vi "Dresden R2R Sputter 03.02.2018 IY24.vi"() -> ()   [LabVIEW 2009] (continued)
                                }
                                frame #1 {
                                }
                                }
                                }
                                frame #1 {
                                n25584 = local read "Semi"() -> (w30862:bool)
                                n25585 = case shown="False" w30862 {
                                frame #0 {
                                n25586 = while {
                                i -> [w30872]
                                stop <- w30863 stop-if-true
                                n25587 = Greater Or Equal?(x=w30872, y=240) -> (x >= y?=w30871:bool)
                                n25588 = case shown="True" w30871 {
                                frame #0 {
                                }
                                frame #1 {
                                n25589 = local write "Semi"(TRUE ("Semi")) -> ()
                                }
                                }
                                n25590 = local read "Set DC Power       :"() -> (w30868:dbl)
                                n25591 = local read "Actual DC Power"() -> (w30867:dbl)
                                n25592 = Subtract(x=w30868, y=w30867) -> (x-y=w30870:dbl)
                                n25593 = Less?(x=w30870, y=10.0) -> (x < y?=w30865:bool)
                                n25594 = local read "Semi"() -> (w30864:bool)
                                n25595 = Or(x=w30865, y=w30864) -> (x .or. y?=w30863:bool)
                                n25596 = Wait Until Next ms Multiple(millisecond multiple=u32 500) -> ()  [unwired: 1 out]
                                }
                                }
                                frame #1 {
                                }
                                }
                                }
                                }
                                }
                                frame #3 {
                                # "Set Pressure for coating"
                                n25597 = stacked-sequence {
                                frame #0 {
                                n25598 = local read "Semi"() -> (w30875:bool)
                                n25599 = case shown="False" w30875 {
                                frame #0 {
                                n25600 = stacked-sequence {
                                frame #0 {
                                n25601 = local read "Semi"() -> (w30876:bool)
                                n25602 = case shown="False" w30876 {
                                frame #0 {
                                n25603 = local read "R Set Pressure mtorr"() -> (w30877:dbl)
                                n25604 = local write "Set_pressure_value 2"(w30877) -> ()
                                }
                                frame #1 {
                                }
                                }
                                }
                                frame #1 {
                                n25605 = local read "Semi"() -> (w30878:bool)
                                n25606 = case shown="False" w30878 {
                                frame #0 {
                                n25607 = Wait (ms)(milliseconds to wait=u32 200) -> ()  [unwired: 1 out]
                                }
                                frame #1 {
                                }
                                }
                                }
                                frame #2 {
                                n25608 = local read "Semi"() -> (w30880:bool)
                                n25609 = case shown="False" w30880 {
                                frame #0 {
                                n25610 = local write "Pc_bv2_auto_set_pressure"(TRUE ("Pc_bv1_auto_set_pressure")) -> ()
                                }
                                frame #1 {
                                }
                                }
                                }
                                frame #3 {
                                n25611 = local read "Semi"() -> (w30882:bool)
                                n25612 = case shown="False" w30882 {
                                frame #0 {
                                n25613 = while {
                                i -> [w30893]
                                stop <- w30885 stop-if-true
                                n25614 = local read "Set_pressure_value 2"() -> (w30883:dbl)
                                n25615 = Greater?(x=w30893, y=300) -> (0:w30887:bool)
                                n25616 = Add(x=1.0, y=w30883) -> (x+y=w30889:dbl)
                                n25617 = Subtract(x=w30883, y=1.0) -> (x-y=w30890:dbl)
                                n25618 = local read "Pressure 2"() -> (w30884:i32)
                                n25619 = In Range and Coerce(upper limit=w30889, x=w30884, lower limit=w30890) -> (In Range?=w30888:bool)  [unwired: 1 out]
                                n25620 = case shown="False" w30888 {
                                tunnel: [FALSE TRUE] -> w30886
                                frame #0 {
                                n25621 = Wait Until Next ms Multiple(millisecond multiple=u32 200) -> ()  [unwired: 1 out]
                                }
                                frame #1 {
                                }
                                }
                                n25622 = Or(x=w30886, y=w30887) -> (x .or. y?=w30885:bool)
                                }
                                }
                                frame #1 {
                                }
                                }
                                }
                                frame #4 {
                                n25623 = local read "Semi"() -> (w30898:bool)
                                n25624 = case shown="False" w30898 {
                                frame #0 {
                                n25625 = local read "Set_pressure_value 2"() -> (w30899:dbl)
                                n25626 = Add(x=1.0, y=w30899) -> (x+y=w30902:dbl)
                                n25627 = Subtract(x=w30899, y=1.0) -> (x-y=w30903:dbl)
                                n25628 = local read "Pressure 2"() -> (w30900:i32)
                                n25629 = In Range and Coerce(upper limit=w30902, x=w30900, lower limit=w30903) -> (In Range?=w30901:bool)  [unwired: 1 out]
                                n25630 = case shown="False" w30901 {
                                frame #0 {
                                n25631 = local read "R Set Pressure mtorr"() -> (w30906:dbl)
                                n25632 = local write "Set_pressure_value 2"(w30906) -> ()
                                }
                                frame #1 {
                                }
                                }
                                }
                                frame #1 {
                                }
                                }
                                }
                                frame #5 {
                                n25633 = local read "Semi"() -> (w30907:bool)
                                n25634 = case shown="False" w30907 {
                                frame #0 {
                                n25635 = local read "Set_pressure_value 2"() -> (w30908:dbl)
                                n25636 = Add(x=1.0, y=w30908) -> (x+y=w30911:dbl)
                                n25637 = Subtract(x=w30908, y=1.0) -> (x-y=w30912:dbl)
                                n25638 = local read "Pressure 2"() -> (w30909:i32)
                                n25639 = In Range and Coerce(upper limit=w30911, x=w30909, lower limit=w30912) -> (In Range?=w30910:bool)  [unwired: 1 out]
                                n25640 = case shown="False" w30910 {
                                frame #0 {
                                n25641 = local write "Pc_bv2_auto_set_pressure"(TRUE ("Pc_bv1_auto_set_pressure")) -> ()
                                }
                                frame #1 {
                                }
                                }
                                }
                                frame #1 {
                                }
                                }
                                }
                                frame #6 {
                                n25642 = local read "Semi"() -> (w30916:bool)
                                n25643 = case shown="False" w30916 {
                                frame #0 {
                                n25644 = while {
                                i -> [w30927]
                                stop <- w30918 stop-if-true
                                n25645 = local read "Set_pressure_value 2"() -> (w30922:dbl)
                                n25646 = Greater?(x=w30927, y=300) -> (0:w30920:bool)
                                n25647 = Add(x=1.0, y=w30922) -> (x+y=w30923:dbl)
                                n25648 = Subtract(x=w30922, y=1.0) -> (x-y=w30924:dbl)
                                n25649 = local read "Pressure 2"() -> (w30917:i32)
                                n25650 = In Range and Coerce(upper limit=w30923, x=w30917, lower limit=w30924) -> (In Range?=w30921:bool)  [unwired: 1 out]
                                n25651 = case shown="False" w30921 {
                                tunnel: [FALSE TRUE] -> w30919
                                frame #0 {
                                n25652 = Wait Until Next ms Multiple(millisecond multiple=u32 200) -> ()  [unwired: 1 out]
                                }
                                frame #1 {
                                }
                                }
                                n25653 = Or(x=w30919, y=w30920) -> (x .or. y?=w30918:bool)
                                }
                                }
                                frame #1 {
                                }
                                }
                                }
                                frame #7 {
                                n25654 = local read "Semi"() -> (w30932:bool)
                                n25655 = case shown="False" w30932 {
                                frame #0 {
                                n25656 = local read "Set_pressure_value 2"() -> (w30935:dbl)
                                n25657 = Add(x=1.0, y=w30935) -> (x+y=w30936:dbl)
                                n25658 = Subtract(x=w30935, y=1.0) -> (x-y=w30937:dbl)
                                n25659 = local read "Pressure 2"() -> (w30933:i32)
                                n25660 = In Range and Coerce(upper limit=w30936, x=w30933, lower limit=w30937) -> (In Range?=w30934:bool)  [unwired: 1 out]
                                n25661 = case shown="False" w30934 {
                                frame #0 {
                                n25662 = local write "Semi"(TRUE ("Semi")) -> ()
                                n25663 = local write "Error Message"("Coating Pressure could not be adjusted !" ("Error Message")) -> ()
                                }
                                frame #1 {
                                }
                                }
                                }
                                frame #1 {
                                }
                                }
                                }
                                }
                                }
                                frame #1 {
                                }
                                }
                                }
                                frame #1 {
                                n25664 = local read "Semi"() -> (w30942:bool)
                                n25665 = case shown="False" w30942 {
                                frame #0 {
                                n25666 = local write "SDC1 9"(TRUE ("SDC1 9")) -> ()
                                n25667 = Wait (ms)(milliseconds to wait=u32 1000) -> ()  [unwired: 1 out]
                                }
                                frame #1 {
                                }
                                }
                                }
                                }
                                }
                                }
                                }
                                frame #1 {
                                }
                                }
                                }
                                frame #11 {
                                n25668 = local read "Semi"() -> (w30945:bool)
                                n25669 = case shown="False" w30945 {
                                frame #0 {
                                n25670 = local write "Start_roll"(TRUE ("Start_roll")) -> ()
                                n25671 = Wait (ms)(milliseconds to wait=u32 300) -> ()  [unwired: 1 out]
                                }
                                frame #1 {
                                }
                                }
                                }
                                frame #12 {
                                n25672 = local read "Semi"() -> (w30948:bool)
                                n25673 = case shown="False" w30948 {
                                frame #0 {
                                n25674 = stacked-sequence {
                                frame #0 {
                                n25675 = local read "R Single DC Step1 Coating Power Active"() -> (w30949:bool)
                                n25676 = case shown="True" w30949 {
                                frame #0 {
                                }
                                frame #1 {
                                n25677 = while {
                                stop <- w30951 stop-if-true
                                n25678 = local read "R Single DC Interval length"() -> (w30955:dbl)
                                n25679 = local read "Actual Length"() -> (w30954:dbl)
                                n25680 = Greater Or Equal?(x=w30954, y=w30955) -> (x >= y?=w30953:bool)
                                n25681 = local read "Semi"() -> (w30952:bool)
                                n25682 = Or(x=w30953, y=w30952) -> (x .or. y?=w30951:bool)
                                n25683 = Wait Until Next ms Multiple(millisecond multiple=u32 300) -> ()  [unwired: 1 out]
                                }
                                }
                                }
                                }
                                frame #1 {
                                n25684 = local read "R Single DC Step2 Coating Power Active"() -> (w30956:bool)
                                n25685 = case shown="True" w30956 {
                                frame #0 {
                                }
                                frame #1 {
                                n25686 = stacked-sequence {
                                frame #0 {
                                n25687 = local read "Semi"() -> (w30957:bool)
                                n25688 = case shown="False" w30957 {
                                frame #0 {
                                n25689 = local read "R Single DC Step2 Coating Power"() -> (w30959:dbl)
                                n25690 = Wait (ms)(milliseconds to wait=u32 200) -> ()  [unwired: 1 out]
                                n25691 = local write "Set DC Power       :"(w30959) -> ()
                                }
                                frame #1 {
                                }
                                }
                                }
                                frame #1 {
                                n25692 = local read "Semi"() -> (w30960:bool)
                                n25693 = case shown="False" w30960 {
                                frame #0 {
                                n25694 = local write "Dc_auto_set"(TRUE ("Dc_auto_set")) -> ()
                                }
                                frame #1 {
                                }
                                }
                                }
                                frame #2 {
                                n25695 = while {
                                stop <- w30966 stop-if-true
                                n25696 = local read "R Single DC Interval length"() -> (w30965:dbl)
                                n25697 = local read "Actual Length"() -> (w30969:dbl)
                                n25698 = Multiply(x=w30965, y=2.0) -> (x*y=w30963:dbl)
                                n25699 = Greater Or Equal?(x=w30969, y=w30963) -> (x >= y?=w30968:bool)
                                n25700 = local read "Semi"() -> (w30967:bool)
                                n25701 = Or(x=w30968, y=w30967) -> (x .or. y?=w30966:bool)
                                n25702 = Wait Until Next ms Multiple(millisecond multiple=u32 300) -> ()  [unwired: 1 out]
                                }
                                }
                                }
                                }
                                }
                                }
                                frame #2 {
                                n25703 = local read "R Single DC Step3 Coating Power Active"() -> (w30970:bool)
                                n25704 = case shown="True" w30970 {
                                frame #0 {
                                }
                                frame #1 {
                                n25705 = stacked-sequence {
                                frame #0 {
                                n25706 = local read "Semi"() -> (w30971:bool)
                                n25707 = case shown="False" w30971 {
                                frame #0 {
                                n25708 = local read "R Single DC Step3 Coating Power"() -> (w30973:dbl)
                                n25709 = Wait (ms)(milliseconds to wait=u32 200) -> ()  [unwired: 1 out]
                                n25710 = local write "Set DC Power       :"(w30973) -> ()
                                }
                                frame #1 {
                                }
                                }
                                }
                                frame #1 {
                                n25711 = local read "Semi"() -> (w30974:bool)
                                n25712 = case shown="False" w30974 {
                                frame #0 {
                                n25713 = local write "Dc_auto_set"(TRUE ("Dc_auto_set")) -> ()
                                }
                                frame #1 {
                                }
                                }
                                }
                                frame #2 {
                                n25714 = while {
                                stop <- w30980 stop-if-true
                                n25715 = local read "R Single DC Interval length"() -> (w30979:dbl)
                                n25716 = local read "Actual Length"() -> (w30983:dbl)
                                n25717 = Multiply(x=w30979, y=3.0) -> (x*y=w30977:dbl)
                                n25718 = Greater Or Equal?(x=w30983, y=w30977) -> (x >= y?=w30982:bool)
                                n25719 = local read "Semi"() -> (w30981:bool)
                                n25720 = Or(x=w30982, y=w30981) -> (x .or. y?=w30980:bool)
                                n25721 = Wait Until Next ms Multiple(millisecond multiple=u32 300) -> ()  [unwired: 1 out]
                                }
                                }
                                }
                                }
                                }
                                }
                                frame #3 {
                                n25722 = local read "R Single DC Step4 Coating Power Active"() -> (w30984:bool)
                                n25723 = case shown="True" w30984 {
                                frame #0 {
                                }
                                frame #1 {
                                n25724 = stacked-sequence {
                                frame #0 {
                                n25725 = local read "Semi"() -> (w30985:bool)
                                n25726 = case shown="False" w30985 {
                                frame #0 {
                                n25727 = local read "R Single DC Step4 Coating Power"() -> (w30987:dbl)
                                n25728 = Wait (ms)(milliseconds to wait=u32 200) -> ()  [unwired: 1 out]
                                n25729 = local write "Set DC Power       :"(w30987) -> ()
                                }
                                frame #1 {
                                }
                                }
                                }
                                frame #1 {
                                n25730 = local read "Semi"() -> (w30988:bool)
                                n25731 = case shown="False" w30988 {
                                frame #0 {
                                n25732 = local write "Dc_auto_set"(TRUE ("Dc_auto_set")) -> ()
                                }
                                frame #1 {
                                }
                                }
                                }
                                frame #2 {
                                n25733 = while {
                                stop <- w30994 stop-if-true
                                n25734 = local read "R Single DC Interval length"() -> (w30993:dbl)
                                n25735 = local read "Actual Length"() -> (w30997:dbl)
                                n25736 = Multiply(x=w30993, y=4.0) -> (x*y=w30991:dbl)
                                n25737 = Greater Or Equal?(x=w30997, y=w30991) -> (x >= y?=w30996:bool)
                                n25738 = local read "Semi"() -> (w30995:bool)
                                n25739 = Or(x=w30996, y=w30995) -> (x .or. y?=w30994:bool)
                                n25740 = Wait Until Next ms Multiple(millisecond multiple=u32 300) -> ()  [unwired: 1 out]
                                }
                                }
                                }
                                }
                                }
                                }
                                frame #4 {
                                n25741 = local read "R Single DC Step5 Coating Power Active"() -> (w30998:bool)
                                n25742 = case shown="True" w30998 {
                                frame #0 {
                                }
                                frame #1 {
                                n25743 = stacked-sequence {
                                frame #0 {
                                n25744 = local read "Semi"() -> (w30999:bool)
                                n25745 = case shown="False" w30999 {
                                frame #0 {
                                n25746 = local read "R Single DC Step5 Coating Power"() -> (w31001:dbl)
                                n25747 = Wait (ms)(milliseconds to wait=u32 200) -> ()  [unwired: 1 out]
                                n25748 = local write "Set DC Power       :"(w31001) -> ()
                                }
                                frame #1 {
                                }
                                }
                                }
                                frame #1 {
                                n25749 = local read "Semi"() -> (w31002:bool)
                                n25750 = case shown="False" w31002 {
                                frame #0 {
                                n25751 = local write "Dc_auto_set"(TRUE ("Dc_auto_set")) -> ()
                                }
                                frame #1 {
                                }
                                }
                                }
                                frame #2 {
                                n25752 = while {
                                stop <- w31008 stop-if-true
                                n25753 = local read "R Single DC Interval length"() -> (w31007:dbl)
                                n25754 = local read "Actual Length"() -> (w31011:dbl)
                                n25755 = Multiply(x=w31007, y=5.0) -> (x*y=w31005:dbl)
                                n25756 = Greater Or Equal?(x=w31011, y=w31005) -> (x >= y?=w31010:bool)
                                n25757 = local read "Semi"() -> (w31009:bool)
                                n25758 = Or(x=w31010, y=w31009) -> (x .or. y?=w31008:bool)
                                n25759 = Wait Until Next ms Multiple(millisecond multiple=u32 300) -> ()  [unwired: 1 out]
                                }
                                }
                                }
                                }
                                }
                                }
                                }
                                }
                                frame #1 {
                                }
                                }
                                }
                                frame #13 {
                                n25760 = local read "Semi"() -> (w31012:bool)
                                n25761 = case shown="False" w31012 {
                                frame #0 {
                                n25762 = local write "SDC1 13b"(TRUE ("SDC1 13b")) -> ()
                                n25763 = Wait (ms)(milliseconds to wait=u32 1000) -> ()  [unwired: 1 out]
                                }
                                frame #1 {
                                }
                                }
                                }
                                }
                                }
                                frame #1 {
                                }
                                }
                                }
                                frame #17 {
                                # "encoder info  add to other web selection"
                                n25764 = stacked-sequence {
                                frame #0 {
                                n25765 = local read "Semi"() -> (w31015:bool)
                                n25766 = case shown="False" w31015 {
                                frame #0 {
                                # "salinim hareketi"
                                n25767 = local read "R_Web_selection"() -> (w31016:enum32{"Web", "Other"})
                                n25768 = case shown="\"Other\"" w31016 {
                                frame #0 {
                                # "TC -ROLL"
                                }
                                frame #1 {
                                n25769 = disable-structure shown="Disabled" {
                                frame #0 {
                                # "OTHER"
                                n25770 = local read "Semi"() -> (w31017:bool)
                                n25771 = case shown="False" w31017 {
                                frame #0 {
                                n25772 = stacked-sequence {
                                frame #0 {
                                n25773 = local read "Semi"() -> (w31018:bool)
                                n25774 = case shown="False" w31018 {
                                frame #0 {
                                n25775 = stacked-sequence {
                                frame #0 {
                                n25776 = local read "Semi"() -> (w31019:bool)
                                n25777 = case shown="False" w31019 {
                                frame #0 {
                                n25778 = while {
                                i -> [w31022]
                                stop <- w31023 stop-if-true
                                n25779 = Greater?(x=w31022, y=300) -> (0:w31020:bool)
                                n25780 = case shown="True" w31020 {
                                frame #0 {
                                }
                                frame #1 {
                                n25781 = local write "Semi"(TRUE ("Semi")) -> ()
                                }
                                }
                                n25782 = local read "RC_13"() -> (w31026:bool)
                                n25783 = case shown="False" w31026 {
                                tunnel: [FALSE ("ch2_1") TRUE ("ch2_1")] -> w31025
                                frame #0 {
                                n25784 = local write "Routine_check_transfer"(TRUE ("ch2_1")) -> ()
                                n25785 = Wait Until Next ms Multiple(millisecond multiple=u32 1000) -> ()  [unwired: 1 out]
                                }
                                frame #1 {
                                }
                                }
                                n25786 = local read "Semi"() -> (w31024:bool)
                                n25787 = Or(x=w31025, y=w31024) -> (x .or. y?=w31023:bool)
                                }
                                }
                                frame #1 {
                                }
                                }
                                }
                                frame #1 {
                                n25788 = local read "Semi"() -> (w31032:bool)
                                n25789 = case shown="False" w31032 {
                                frame #0 {
                                n25790 = while {
                                i -> [w31039]
                                stop <- w31034 stop-if-true
                                n25791 = Greater?(x=w31039, y=100) -> (0:w31037:bool)
                                n25792 = case shown="True" w31037 {
                                frame #0 {
                                }
                                frame #1 {
                                n25793 = local write "Error Message"("Transfer process was cancelled.\nPlease check GV connections." ("Error Message")) -> ()
                                n25794 = local write "Semi"(TRUE ("Semi")) -> ()
                                }
                                }
                                n25795 = local read "Ch1_Trns_interlock_di"() -> (w31033:bool)
                                n25796 = case shown="False" w31033 {
                                tunnel: [w31041 TRUE] -> w31036
                                frame #0 {
                                n25797 = local read "Ch1_TGV_control_di"() -> (w31040:bool)
                                n25798 = case shown="False" w31040 {
                                tunnel: [FALSE TRUE] -> w31041
                                frame #0 {
                                n25799 = Wait Until Next ms Multiple(millisecond multiple=u32 50) -> ()  [unwired: 1 out]
                                n25800 = local write "Ch1_TGV_control_do"(TRUE ("Ch1_pet_cool_up_do")) -> ()
                                }
                                frame #1 {
                                }
                                }
                                }
                                frame #1 {
                                }
                                }
                                n25801 = local read "Semi"() -> (w31035:bool)
                                n25802 = Or(x=w31036, y=w31035) -> (x .or. y?=w31034:bool)
                                }
                                }
                                frame #1 {
                                }
                                }
                                }
                                frame #2 {
                                n25803 = local read "Semi"() -> (w31049:bool)
                                n25804 = case shown="False" w31049 {
                                frame #0 {
                                n25805 = while {
                                i -> [w31056]
                                stop <- w31051 stop-if-true
                                n25806 = Greater?(x=w31056, y=100) -> (0:w31054:bool)
                                n25807 = case shown="True" w31054 {
                                frame #0 {
                                }
                                frame #1 {
                                n25808 = local write "Error Message"("Transfer process was cancelled.\nPlease check GV connections." ("Error Message")) -> ()
                                n25809 = local write "Semi"(TRUE ("Semi")) -> ()
                                }
                                }
                                n25810 = local read "Ch2_Trns_interlock_di"() -> (w31050:bool)
                                n25811 = case shown="False" w31050 {
                                tunnel: [w31058 TRUE] -> w31053
                                frame #0 {
                                n25812 = local read "Ch2_TGV_control_di"() -> (w31057:bool)
                                n25813 = case shown="False" w31057 {
                                tunnel: [FALSE TRUE] -> w31058
                                frame #0 {
                                n25814 = Wait Until Next ms Multiple(millisecond multiple=u32 50) -> ()  [unwired: 1 out]
                                n25815 = local write "Ch2_TGV_control_do"(TRUE ("Ch1_pet_cool_up_do")) -> ()
                                }
                                frame #1 {
                                }
                                }
                                }
                                frame #1 {
                                }
                                }
                                n25816 = local read "Semi"() -> (w31052:bool)
                                n25817 = Or(x=w31053, y=w31052) -> (x .or. y?=w31051:bool)
                                }
                                }
                                frame #1 {
                                }
                                }
                                }
                                frame #3 {
                                n25818 = local read "Semi"() -> (w31066:bool)
                                n25819 = case shown="False" w31066 {
                                frame #0 {
                                n25820 = while {
                                i -> [w31073]
                                stop <- w31068 stop-if-true
                                n25821 = Greater?(x=w31073, y=100) -> (0:w31071:bool)
                                n25822 = case shown="True" w31071 {
                                frame #0 {
                                }
                                frame #1 {
                                n25823 = local write "Error Message"("Transfer process was cancelled.\nPlease check GV connections." ("Error Message")) -> ()
                                n25824 = local write "Semi"(TRUE ("Semi")) -> ()
                                }
                                }
                                n25825 = local read "Ch3_Trns_interlock_di"() -> (w31067:bool)
                                n25826 = case shown="False" w31067 {
                                tunnel: [w31075 TRUE] -> w31070
                                frame #0 {
                                n25827 = local read "Ch3_TGV_control_di"() -> (w31074:bool)
                                n25828 = case shown="False" w31074 {
                                tunnel: [FALSE TRUE] -> w31075
                                frame #0 {
                                n25829 = Wait Until Next ms Multiple(millisecond multiple=u32 50) -> ()  [unwired: 1 out]
                                n25830 = local write "Ch3_TGV_control_do"(TRUE ("Ch1_pet_cool_up_do")) -> ()
                                }
                                frame #1 {
                                }
                                }
                                }
                                frame #1 {
                                }
                                }
                                n25831 = local read "Semi"() -> (w31069:bool)
                                n25832 = Or(x=w31070, y=w31069) -> (x .or. y?=w31068:bool)
                                }
                                }
                                frame #1 {
                                }
                                }
                                }
                                frame #4 {
                                n25833 = local read "Semi"() -> (w31083:bool)
                                n25834 = case shown="False" w31083 {
                                frame #0 {
                                n25835 = while {
                                i -> [w31090]
                                stop <- w31085 stop-if-true
                                n25836 = Greater?(x=w31090, y=100) -> (0:w31088:bool)
                                n25837 = case shown="True" w31088 {
                                frame #0 {
                                }
                                frame #1 {
                                n25838 = local write "Error Message"("Transfer process was cancelled.\nPlease check GV connections." ("Error Message")) -> ()
                                n25839 = local write "Semi"(TRUE ("Semi")) -> ()
                                }
                                }
                                n25840 = local read "Ch3_Trns_interlock_di"() -> (w31084:bool)
                                n25841 = case shown="False" w31084 {
                                tunnel: [w31092 TRUE] -> w31087
                                frame #0 {
                                n25842 = local read "Ch3_TGV_control_di"() -> (w31091:bool)
                                n25843 = case shown="False" w31091 {
                                tunnel: [FALSE TRUE] -> w31092
                                frame #0 {
                                n25844 = Wait Until Next ms Multiple(millisecond multiple=u32 50) -> ()  [unwired: 1 out]
                                n25845 = local write "Ch3_TGV_control_do"(TRUE ("Ch1_pet_cool_up_do")) -> ()
                                }
                                frame #1 {
                                }
                                }
                                }
                                frame #1 {
                                }
                                }
                                n25846 = local read "Semi"() -> (w31086:bool)
                                n25847 = Or(x=w31087, y=w31086) -> (x .or. y?=w31085:bool)
                                }
                                }
                                frame #1 {
                                }
                                }
                                }
                                frame #5 {
                                n25848 = local read "Semi"() -> (w31100:bool)
                                n25849 = case shown="False" w31100 {
                                frame #0 {
                                n25850 = while {
                                i -> [w31103]
                                stop <- w31104 stop-if-true
                                n25851 = Greater?(x=w31103, y=50) -> (0:w31101:bool)
                                n25852 = case shown="True" w31101 {
                                frame #0 {
                                }
                                frame #1 {
                                n25853 = local write "Error Message"("Transfer process was\ncancelled.Please check right slow sensor." ("Error Message")) -> ()
                                n25854 = local write "Semi"(TRUE ("Semi")) -> ()
                                }
                                }
                                n25855 = local read "Cnt_Right_slow_di"() -> (w31107:bool)
                                n25856 = case shown="False" w31107 {
                                tunnel: [FALSE ("Ch1_pet_cool_up_do") TRUE ("Ch1_pet_cool_up_do")] -> w31106
                                frame #0 {
                                n25857 = local write "Cnt_Right_slow_do"(TRUE ("Ch1_pet_cool_up_do")) -> ()
                                n25858 = Wait Until Next ms Multiple(millisecond multiple=u32 200) -> ()  [unwired: 1 out]
                                }
                                frame #1 {
                                }
                                }
                                n25859 = local read "Semi"() -> (w31105:bool)
                                n25860 = Or(x=w31106, y=w31105) -> (x .or. y?=w31104:bool)
                                }
                                }
                                frame #1 {
                                }
                                }
                                }
                                frame #6 {
                                n25861 = local read "Semi"() -> (w31114:bool)
                                n25862 = case shown="False" w31114 {
                                frame #0 {
                                n25863 = while {
                                i -> [w31115]
                                stop <- w31119 stop-if-true
                                n25864 = Greater?(x=w31115, y=50) -> (0:w31117:bool)
                                n25865 = case shown="True" w31117 {
                                frame #0 {
                                }
                                frame #1 {
                                n25866 = local write "Error Message"("Transfer process was\ncancelled.Please check right limit sensor." ("Error Message")) -> ()
                                n25867 = local write "Semi"(TRUE ("Semi")) -> ()
                                }
                                }
                                n25868 = local read "Cnt_Right_limit_di"() -> (w31121:bool)
                                n25869 = case shown="False" w31121 {
                                tunnel: [FALSE ("Ch1_pet_cool_up_do") TRUE ("Ch1_pet_cool_up_do")] -> w31120
                                frame #0 {
                                n25870 = local write "Cnt_Right_limit_do"(TRUE ("Ch1_pet_cool_up_do")) -> ()
                                n25871 = Wait Until Next ms Multiple(millisecond multiple=u32 200) -> ()  [unwired: 1 out]
                                }
                                frame #1 {
                                }
                                }
                                n25872 = local read "Semi"() -> (w31118:bool)
                                n25873 = Or(x=w31120, y=w31118) -> (x .or. y?=w31119:bool)
                                }
                                }
                                frame #1 {
                                }
                                }
                                }
                                frame #7 {
                                n25874 = local read "Semi"() -> (w31128:bool)
                                n25875 = case shown="False" w31128 {
                                frame #0 {
                                n25876 = while {
                                i -> [w31131]
                                stop <- w31132 stop-if-true
                                n25877 = Greater?(x=w31131, y=50) -> (0:w31129:bool)
                                n25878 = case shown="True" w31129 {
                                frame #0 {
                                }
                                frame #1 {
                                n25879 = local write "Error Message"("Transfer process was\ncancelled.Please check left slow sensor." ("Error Message")) -> ()
                                n25880 = local write "Semi"(TRUE ("Semi")) -> ()
                                }
                                }
                                n25881 = local read "Cnt_Left_slow_di"() -> (w31135:bool)
                                n25882 = case shown="False" w31135 {
                                tunnel: [FALSE ("Ch1_pet_cool_up_do") TRUE ("Ch1_pet_cool_up_do")] -> w31134
                                frame #0 {
                                n25883 = local write "Cnt_Left_slow_do"(TRUE ("Ch1_pet_cool_up_do")) -> ()
                                n25884 = Wait Until Next ms Multiple(millisecond multiple=u32 200) -> ()  [unwired: 1 out]
                                }
                                frame #1 {
                                }
                                }
                                n25885 = local read "Semi"() -> (w31133:bool)